vi "labHolo.vi"() -> ()   [LabVIEW 2023] (continued)
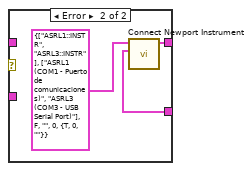
[diagram p2: hidden frame]
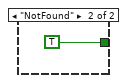
[diagram p4: hidden frame]
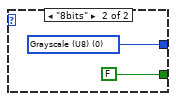
[diagram p5: hidden frame]
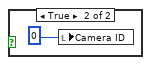
[diagram p6: hidden frame]
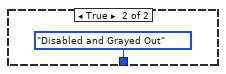
[diagram p7: hidden frame]
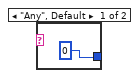
[diagram p13: hidden frame]
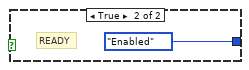
[diagram p14: hidden frame]
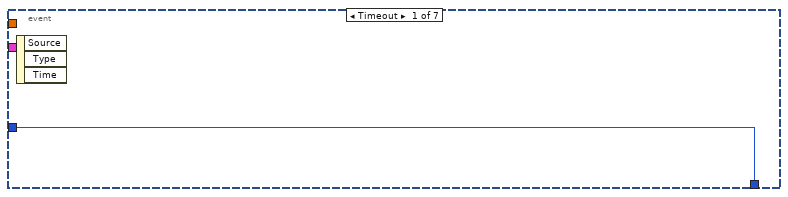
[diagram p15: hidden frame]
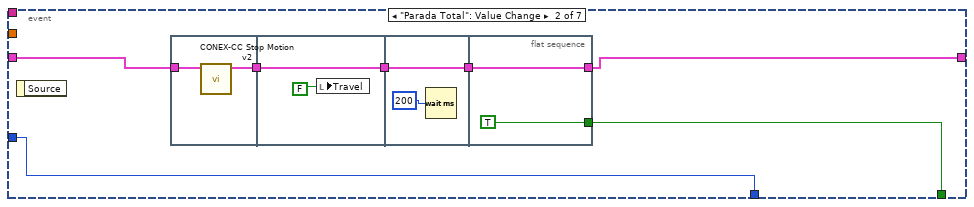
[diagram p16: hidden frame]
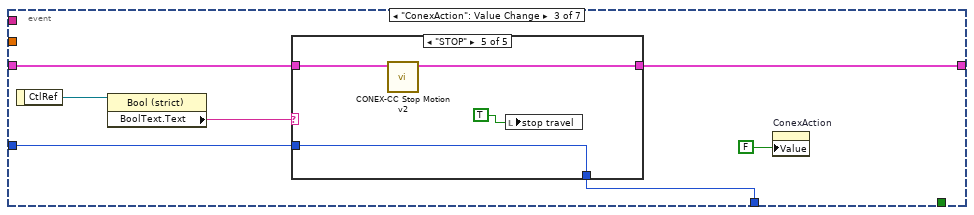
[diagram p17: hidden frame]
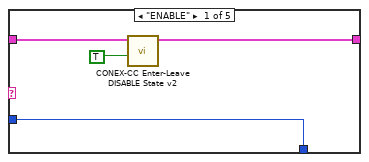
[diagram p18: hidden frame]
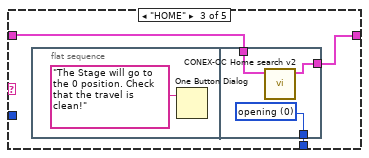
[diagram p20: hidden frame]
            n224 = local write "take reff"(w850) -> ()
            n225 = local write "Mean array"(w851) -> ()
            n226 = local write "Var array"(w851) -> ()
          }
          event "suffix", "Polarizer", "Analyzer", "beam_name", "Save": Value Change {
            n227 = event-data() -> ("CtlRef"=w866:refnum<vi>)  [unwired: 1 in, 5 out]
            n228 = local read "Travel"() -> (w853:bool)
            n229 = property class="Ctl"(reference=w866, error in=w860) -> (reference out=w861:refnum<vi>, error out=w859:errorcluster, "Label.Text"=w865:string)
            n230 = local read "beam_name"() -> (w870:string)
            n231 = local read "paramAux"() -> (w867:string)
            n232 = case shown="True" w853 {
              tunnel: w855 -> [_ w873]
              tunnel: [w871 w872] -> w854
              frame False {
                n233 = local read "suffix"() -> (w871:string)
              }
              frame True {
                n234 = Wait on Notification with Notifier History(0:w873) -> (9:w872:string)  [unwired: 3 in, 3 out]
                n235 = local write "suffix"(w872) -> ()
              }
            }
            n236 = local read "Polarizer"() -> (w869:string)
            n237 = local read "Analyzer"() -> (w868:string)
            n238 = call "getSavePath.vi"("beam_name"=w870, "Polarizer"=w869, "Analyzer"=w868, "prefix"=w867, "suffix"=w854) -> ("appended filename"=w858:string)  [unwired: 10 in]
            n239 = case shown="\"Save\"" w865 {
              tunnel: w858 -> [w874 w891]
              tunnel: w864 -> [_ w893]
              tunnel: w863 -> [_ w892]
              tunnel: [errorcluster {"status"=FALSE, "code"=0, "source"=""} ("error out") w881] -> w862
              tunnel: w861 -> [_ w885]
              tunnel: w859 -> [_ w886]
              tunnel: [w874 w887] -> w856
              tunnel: w853 -> [_ w877]
              frame "Any", Default {
              }
              frame "Save" {
                n240 = property on="Property Node" class="Ctl"(reference=w885, error in=w886, "DisabledEnum"=T11."Disabled and Grayed Out" ("Disabled")) -> (reference out=w884:refnum<vi>, error out=w883:errorcluster)
                n241 = Not(x=w877) -> (.not. x?=w876:bool)
                n242 = local read "Reff ROI"() -> (w889:T8)
                n243 = local read "bit depth"() -> (w888:enum16{"16bits", "14bits", "12bits", "8bits"})
                n244 = property on="CCD Image" class="ImageControl"() -> ("ROI"=w890:T8)  [unwired: 2 in, 2 out]
                n245 = call "saveImage.vi"("UserDialog"=w876, "error in"=w883, "bit depth"=w888, "session in"=w892, "Reff ROI"=w889, "main ROI"=w890, "appended filename"=w891, "Image in"=w893) -> ("error out"=w882:errorcluster, "png filename"=w887:string)  [unwired: 2 out]
                n246 = property on="Property Node" class="Ctl"(reference=w884, error in=w882, "DisabledEnum"=T11."Enabled" ("Disabled"), "Value"=FALSE ("Save")) -> (error out=w881:errorcluster)  [unwired: 1 out]
              }
            }
            n247 = local write "default filename"(w858) -> ()
            n248 = Send Notification(notification=w856, notifier=w857) -> ()  [unwired: 1 in, 2 out]
          }
          event "FPS", "Exposure (ms)", "Gain": Value Change {
            n249 = event-data() -> ("CtlRef"=w902:refnum<vi>, "NewVal"=w905:dbl)  [unwired: 1 in, 4 out]
            n250 = property class="DigNum (strict)"(reference=w902) -> ("Label.Text"=w903:string)  [unwired: 1 in, 2 out]
            n251 = case shown="\"FPS\"" w903 {
              tunnel: w906 -> [w913 w920 w929]
              tunnel: w905 -> [w912 w919 w921]
              tunnel: [w911 w918 w927] -> w904
              tunnel: w895 -> [w908 w917 w922]
              tunnel: [w909 w916 w926] -> w897
              tunnel: [w910 w915 w925] -> w896
              tunnel: w894 -> [w907 w914 w928]
              frame "Exposure (ms)", Default {
                n252 = call "set_exposure.vi"("error in (no error)"=w907, "cam ID"=w908, "exposure"=w912, "Session in"=w913) -> ("error out"=w911:errorcluster, "true FPS"=w909:dbl, "true exposure"=w910:dbl)  [unwired: 3 in, 1 out]
              }
              frame "FPS" {
                n253 = call "set_fps.vi"("error in (no error)"=w914, "cam ID"=w917, "FPS"=w919, "Session in"=w920) -> ("error out"=w918:errorcluster, "true Exposure"=w915:dbl, "true FPS"=w916:dbl)  [unwired: 3 in, 1 out]
              }
              frame "Gain" {
                n254 = local read "gains"() -> (w924:dbl[])
                n255 = call "set_gain.vi"("error in (no error)"=w928, "cam ID"=w922, "Gain"=w921, "Session in"=w929) -> ("error out"=w927:errorcluster, "true Exposure"=w925:dbl, "true FPS"=w926:dbl)  [unwired: 3 in, 1 out]
                n256 = Replace Array Subset(array=w924, new element=w921, index=w922) -> (w923:dbl[])
                n257 = local write "gains"(w923) -> ()
              }
            }
            n258 = local write "Exposure (ms)"(w896) -> ()
            n259 = local write "FPS"(w897) -> ()
            n260 = local read "exposures"() -> (w900:dbl[])
            n261 = local read "FPSs"() -> (w901:dbl[])
            n262 = Replace Array Subset(array=w900, new element=w896, index=w895) -> (w898:dbl[])
            n263 = Replace Array Subset(array=w901, new element=w897, index=w895) -> (w899:dbl[])
            n264 = local write "exposures"(w898) -> ()
            n265 = local write "FPSs"(w899) -> ()
          }
          event "Camera ID": Value Change {
            n266 = event-data() -> ("OldVal"=w931:u16, "NewVal"=w930:u16)  [unwired: 1 in, 4 out]
            n267 = flat-sequence {
              tunnel: w931 -> [w932]
              tunnel: w930 -> [w944]
              frame #0 {
                n268 = local read "Exposure (ms)"() -> (w941:dbl)
                n269 = local read "gains"() -> (w935:dbl[])
                n270 = local read "FPSs"() -> (w936:dbl[])
                n271 = local read "Gain"() -> (w933:dbl)
                n272 = local read "exposures"() -> (w940:dbl[])
                n273 = local read "FPS"() -> (w938:dbl)
                n274 = Replace Array Subset(array=w935, new element=w933, index=w932) -> (w934:dbl[])
                n275 = Replace Array Subset(array=w940, new element=w941, index=w932) -> (w939:dbl[])
                n276 = Replace Array Subset(array=w936, new element=w938, index=w932) -> (w937:dbl[])
                n277 = local write "exposures"(w939) -> ()
                n278 = local write "FPSs"(w937) -> ()
                n279 = local write "gains"(w934) -> ()
              }
              frame #1 {
                n280 = local read "exposures"() -> (w950:dbl[])
                n281 = local read "FPSs"() -> (w949:dbl[])
                n282 = local read "gains"() -> (w943:dbl[])
                n283 = Index Array(array=w949, index=w944) -> (element=w948:dbl)
                n284 = Index Array(array=w950, index=w944) -> (element=w947:dbl)
                n285 = Index Array(array=w943, index=w944) -> (element=w942:dbl)
                n286 = property on="FPS" class="DigNum (strict)"("Val(Sgnl)"=w948) -> (error out=w946:errorcluster)  [unwired: 2 in, 1 out]
                n287 = property on="Exposure (ms)" class="DigNum (strict)"(error in=w946, "Val(Sgnl)"=w947) -> (error out=w945:errorcluster)  [unwired: 1 in, 1 out]
                n288 = property on="Gain" class="DigNum (strict)"(error in=w945, "Val(Sgnl)"=w942) -> ()  [unwired: 1 in, 2 out]
              }
            }
          }
          event "Parada Total": Value Change {
            n289 = event-data() -> ("NewVal"=w951:bool)  [unwired: 1 in, 5 out]
          }
        }
        "py error" <- w804
      }
      n290 = timed-loop {
        timing: w292 -> [_]
        timing-out: [_] -> w291
        shift-right: [w383] -> w290
        shift-left: w289 -> [w389]
        tunnel: w277 -> [w369]
        stop <- w384 stop-if-true
        # "Working loop"
        n291 = node-c288() -> ()  [unwired: 2 out]
        n292 = call "CONEX-CC Get Current Position v2.vi"("Connection Cluster in"=w389) -> ("Current position"=w380:dbl, "Connection Cluster out"=w388:T16)  [unwired: 8 in, 1 out]
        n293 = local read "Travel"() -> (w373:bool)
        n294 = call "CONEX-CC Get Positioner Error And Controller State v2.vi"("Connection Cluster in"=w388) -> ("Controller state"=w386:string, "Positioner error"=w387:string, "Connection Cluster out"=w383:T16)  [unwired: 8 in]
        n295 = Not(x=w373) -> (.not. x?=w374:bool)
        n296 = call "Get Positioner Error And Controller State Descriptions.vi"("Controller state"=w386, "Positioner error"=w387) -> ("Color"=w392:u32, "Action name"=w377:string, "Controller state description"=→"Controller state description":string, "IsReady?"=w372:bool)  [unwired: 2 out]
        "ConexCC ready" <- w372
        n297 = And(x=w374, y=w372) -> (x .and. y?=w375:bool)
        n298 = property on="ConexAction" class="Bool (strict)"("BoolText.Text"=w377) -> ()  [unwired: 2 in, 2 out]
        n299 = property on="Controller state description" class="Str"("Text.FontColor"=w392) -> ()  [unwired: 2 in, 2 out]
        n300 = case shown="False" w375 {
          tunnel: [T11."Disabled and Grayed Out" ("Disabled") T11."Enabled" ("Disabled")] -> w378
          frame False {
            # "MOVING"
          }
          frame True {
            # "READY"
          }
        }
        n301 = String Length(string=w377) -> (length=w391:i32)
        n302 = case shown="\"DISABLE\"" w377 {
          tunnel: [0 2] -> w376
          frame "Any", Default {
          }
          frame "DISABLE" {
          }
        }
        n303 = Greater Than 0?(x=w391) -> (x > 0?=w390:bool)
        n304 = property on="ConexAction" class="Bool (strict)"("DisabledEnum"=w376, "Visible"=w390) -> ()  [unwired: 2 in, 2 out]
        n305 = property on="Go0" class="Bool (strict)"("Disabled"=w378) -> ()  [unwired: 2 in, 2 out]
        n306 = property on="Go1" class="Bool (strict)"("Disabled"=w378) -> ()  [unwired: 2 in, 2 out]
        n307 = property on="Go2" class="Bool (strict)"("Disabled"=w378) -> ()  [unwired: 2 in, 2 out]
        n308 = property on="Units" class="CmbBox"("Disabled"=w378) -> ()  [unwired: 2 in, 2 out]
        n309 = property on="Tare" class="Bool (strict)"("Disabled"=w378) -> ()  [unwired: 2 in, 2 out]
        n310 = property on="Travel" class="Bool (strict)"("Disabled"=w378) -> ()  [unwired: 2 in, 2 out]
        n311 = property on="step forward" class="Bool (strict)"("Disabled"=w378) -> ()  [unwired: 2 in, 2 out]
        n312 = property on="step backward" class="Bool (strict)"("Disabled"=w378) -> ()  [unwired: 2 in, 2 out]
        n313 = property on="SaveTravel" class="Bool (strict)"("Disabled"=w378) -> ()  [unwired: 2 in, 2 out]
        n314 = local read "Units"() -> (w382:string)
        n315 = local read "lambda"() -> (w381:dbl)
        n316 = call "mm2units.vi"("lambda (nm)"=w381, "target units"=w382, "raw position (mm)"=w380) -> ("position in units"=w379:dbl)  [unwired: 8 in]
        n317 = local read "Zero pos."() -> (w385:dbl)
        n318 = local read "Travel"() -> (w371:bool)
        n319 = local write "Raw position"(w379) -> ()
        n320 = Subtract(x=w379, y=w385) -> (x-y=w370:dbl)
        n321 = local write "Relative pos."(w370) -> ()
        n322 = case shown="True" w371 {
          tunnel: w370 -> [_ w395]
          tunnel: w369 -> [_ w394]
          frame False {
          }
          frame True {
            n323 = Send Notification(notification=w395, notifier=w394) -> ()  [unwired: 1 in, 2 out]
          }
        }
        n324 = local read "Parada Total"() -> (w384:bool)
        n325 = node-c288() -> ()  [unwired: 2 out]
      }
      n326 = while {
        tunnel: w295 -> [w523]
        shift-right: [w522] -> _
        shift-left: w294 -> [w521]
        shift-right: [w520] -> _
        shift-left: w296 -> [w524]
        shift-right: [w519] -> _
        shift-left: _ -> [w518]
        shift-right: [w516] -> _
        shift-left: w293 -> [w517]
        stop <- w525 stop-if-true
        # "SLM control"
        # "CGH path"
        # "Theo"
        # "SLM"
        n327 = event shown="[1] \"Radio\", \"Trans\", \"HoloNum\", \"ModType\", \"Semi\", \"Active\", \"paramVal\", \"paramStr\", \"paramAux\", \"Phase\", \"Flip\": Value Change" {
          selector: _ -> [_ _ _ _ _ _ _]
          dyn-events: _ -> [_ _ _ _ _ _ _]
          timeout: _ -> [_ _ _ _ _ _ _]
          tunnel: w517 -> [w526 w540 w608 w661 w717 _ _]
          tunnel: [_ _ _ _ _ _ w793] -> w525
          tunnel: w524 -> [w528 w543 _ _ _ w754 _]
          tunnel: w523 -> [_ _ _ _ _ _ _]
          tunnel: [_ w538 _ _ _ _ _] -> w522
          tunnel: w521 -> [_ w546 _ _ _ _ _]
          tunnel: [w528 w539 _ _ _ w756 _] -> w520
          tunnel: [w527 w541 _ _ _ w755 _] -> w519
          tunnel: w518 -> [w527 w542 _ _ _ w753 _]
          tunnel: [w526 w540 w608 w661 w717 w752 _] -> w516
          event Timeout {
            n328 = event-data() -> ()  [unwired: 1 in, 3 out]
          }
          event "Radio", "Trans", "HoloNum", "ModType", "Semi", "Active", "paramVal", "paramStr", "paramAux", "Phase", "Flip": Value Change {
            # "Display = #item + 1"
            # "Old"
            # "New"
            n329 = event-data() -> ("CtlRef"=w544:refnum<vi>, "OldVal"=w550:variant, "NewVal"=w545:variant)  [unwired: 1 in]
            n330 = case shown="1" w540 {
              tunnel: [w555 w556] -> w552
              frame 0, Default {
                n331 = local read "SLM1 cluster"() -> (w555:T2)
              }
              frame 1 {
                n332 = local read "SLM2 cluster"() -> (w556:T2)
              }
            }
            n333 = property class="Ctl"(reference=w544) -> ("Label.Text"=w551:string)  [unwired: 1 in, 2 out]
            n334 = call "updateHoloBundle.vi"("NewValue"=w545, "input cluster"=w552, "CtlRef"=w544) -> ("output cluster"=w549:T19)  [unwired: 7 in, 1 out]
            n335 = Increment(x=w540) -> (x+1=w548:u16)
            n336 = call "loadShowHolo.vi"("Display"=w548, "error in (no error)"=w546, "prev. path"=w542, "SLM1 cluster"=w549, "Image in"=w543) -> ("error out"=w538:errorcluster, "path exist"=w547:bool, "appended path"=w541:path, "Image out"=w539:T6)  [unwired: 3 in]
            n337 = case shown="\"Radio\"" w551 {
              tunnel: w550 -> [w558 w564 _ w570 _ w581 w587 w593 _ _]
              tunnel: w545 -> [_ _ _ _ w579 _ _ _ w602 w606]
              tunnel: w547 -> [w557 w563 _ w569 _ w580 w586 w592 _ _]
              frame "HoloNum" {
                n338 = case shown="False" w557 {
                  tunnel: w558 -> [w559 _]
                  frame False {
                    n339 = feedback #1() -> (w560:dbl)  [unwired: 1 in]
                    n340 = Variant To Data(type=w560, Variant=w559) -> (data=w562:dbl)  [unwired: 1 in, 1 out]
                    n341 = property on="HoloNum" class="DigNum (strict)"("Value"=w562) -> ("Value"=w561:dbl)  [unwired: 2 in, 2 out]
                    n342 = feedback-in #1(w561) -> ()
                  }
                  frame True {
                  }
                }
              }
              frame "ParamStr" {
                n343 = case shown="False" w563 {
                  tunnel: w564 -> [w565 _]
                  frame False {
                    n344 = feedback #2() -> (w566:string)  [unwired: 1 in]
                    n345 = Variant To Data(type=w566, Variant=w565) -> (data=w568:string)  [unwired: 1 in, 1 out]
                    n346 = property on="paramStr" class="Str"("Value"=w568) -> ("Value"=w567:string)  [unwired: 2 in, 2 out]
                    n347 = feedback-in #2(w567) -> ()
                  }
                  frame True {
                  }
                }
              }
              frame "Any", Default {
              }
              frame "ParamVal" {
                n348 = case shown="False" w569 {
                  tunnel: w570 -> [w571 _]
                  frame False {
                    n349 = feedback #3() -> (w572:i64)  [unwired: 1 in]
                    n350 = Variant To Data(type=w572, Variant=w571) -> (data=w574:i64)  [unwired: 1 in, 1 out]
                    n351 = property on="paramVal" class="DigNum (strict)"("Value"=w574) -> ("Value"=w573:i64)  [unwired: 2 in, 2 out]
                    n352 = feedback-in #3(w573) -> ()
                  }
                  frame True {
                  }
                }
              }
              frame "Active" {
                n353 = Variant To Data(type=0, Variant=w579) -> (data=w575:i32)  [unwired: 1 in, 1 out]
                n354 = Not Equal?(x=u16 0, y=w575) -> (x != y?=w576:bool)
                n355 = property on="Active" class="Ring (strict)"("Blinking"=w576) -> ()  [unwired: 2 in, 2 out]
              }
              frame "ParamAux" {
                n356 = case shown="False" w580 {
                  tunnel: w581 -> [w582 _]
                  frame False {
                    n357 = feedback #4() -> (w583:string)  [unwired: 1 in]
                    n358 = Variant To Data(type=w583, Variant=w582) -> (data=w585:string)  [unwired: 1 in, 1 out]
                    n359 = property on="paramAux" class="Str"("Value"=w585) -> ("Value"=w584:string)  [unwired: 2 in, 2 out]
                    n360 = feedback-in #4(w584) -> ()
                  }
                  frame True {
                  }
                }
              }
              frame "ModType" {
                n361 = case shown="False" w586 {
                  tunnel: w587 -> [w589 _]
                  frame False {
                    n362 = feedback #5() -> (w591:string)  [unwired: 1 in]
                    n363 = Variant To Data(type=w591, Variant=w589) -> (data=w588:string)  [unwired: 1 in, 1 out]
                    n364 = property on="ModType" class="CmbBox"("Value"=w588) -> ("Value"=w590:string)  [unwired: 2 in, 2 out]
                    n365 = feedback-in #5(w590) -> ()
                  }
                  frame True {
                  }
                }
              }
              frame "Radio" {
                n366 = case shown="False" w592 {
                  tunnel: w593 -> [w596 _]
                  frame False {
                    n367 = Variant To Data(type=0, Variant=w596) -> (data=w594:i32)  [unwired: 1 in, 1 out]
                    n368 = local write "Radio"(w594) -> ()
                  }
                  frame True {
                  }
                }
              }
              frame "Trans" {
                n369 = Variant To Data(type=0.0, Variant=w602) -> (data=w600:dbl)  [unwired: 1 in, 1 out]
                n370 = call "transAndPhaseManager.vi"("Trans in"=w600) -> ("Trans %"=w599:dbl, "Intensity"=w598:dbl, "T gl"=w597:dbl)  [unwired: 10 in, 2 out]
                n371 = local write "T%"(w599) -> ()
                n372 = local write "Int"(w598) -> ()
                n373 = local write "Tgl"(w597) -> ()
              }
              frame "Phase" {
                n374 = Variant To Data(type=0.0, Variant=w606) -> (data=w603:dbl)  [unwired: 1 in, 1 out]
                n375 = call "transAndPhaseManager.vi"("Phase in"=w603) -> ("Phase Deg"=w605:dbl, "Phase Rad"=w604:dbl)  [unwired: 10 in, 3 out]
                n376 = local write "PhDeg"(w605) -> ()
                n377 = local write "PhRad"(w604) -> ()
              }
            }
            n378 = case shown="1" w540 {
              tunnel: w549 -> [w553 w554]
              frame 0, Default {
                n379 = local write "SLM1 cluster"(w553) -> ()
              }
              frame 1 {
                n380 = local write "SLM2 cluster"(w554) -> ()
              }
            }
            n381 = local read "Radio"() -> (w530:T7)
            n382 = local read "Active"() -> (w537:u16)
            n383 = call "enableDisableSLMbuttons.vi"("Active"=w537, "Radio"=w530) -> ("Semi"=w532:T11, "ModType"=w533:T11, "Phase"=w534:T11, "Trans"=w535:T11, "HoloCode"=w531:T11, "PrefabrHolo"=w536:T11, "just ON/OFF"=w529:T11)  [unwired: 3 in]
            n384 = property on="Flip" class="CmbBox"("DisabledEnum"=w529) -> ()  [unwired: 2 in, 2 out]
            n385 = property on="Radio" class="RadioBtnsControl (strict)"("DisabledEnum"=w529) -> ()  [unwired: 2 in, 2 out]
            n386 = property on="HoloNum" class="DigNum (strict)"("DisabledEnum"=w536) -> ()  [unwired: 2 in, 2 out]
            n387 = property on="paramAux" class="Str"("DisabledEnum"=w536) -> ()  [unwired: 2 in, 2 out]
            n388 = property on="Xoffset" class="DigNum (strict)"("DisabledEnum"=w529) -> ()  [unwired: 2 in, 2 out]
            n389 = property on="Sync SLMs" class="Bool"("DisabledEnum"=w529) -> ()  [unwired: 2 in, 2 out]
            n390 = property on="ModType" class="CmbBox"("DisabledEnum"=w533) -> ()  [unwired: 2 in, 2 out]
            n391 = property on="Trans" class="Slide (strict)"("DisabledEnum"=w535) -> ()  [unwired: 2 in, 2 out]
            n392 = property on="setXi" class="Bool (strict)"("DisabledEnum"=w529) -> ()  [unwired: 2 in, 2 out]
            n393 = property on="paramStr" class="Str"("DisabledEnum"=w536) -> ()  [unwired: 2 in, 2 out]
            n394 = property on="paramVal" class="DigNum (strict)"("DisabledEnum"=w536) -> ()  [unwired: 2 in, 2 out]
            n395 = property on="Yoffset" class="DigNum (strict)"("DisabledEnum"=w529) -> ()  [unwired: 2 in, 2 out]
            n396 = property on="XYswap" class="Ring (strict)"("DisabledEnum"=w529) -> ()  [unwired: 2 in, 2 out]
            n397 = property on="Phase" class="Slide (strict)"("DisabledEnum"=w534) -> ()  [unwired: 2 in, 2 out]
            n398 = property on="T%" class="DigNum (strict)"("DisabledEnum"=w535) -> ()  [unwired: 2 in, 2 out]
            n399 = property on="setXf" class="Bool (strict)"("DisabledEnum"=w529) -> ()  [unwired: 2 in, 2 out]
            n400 = property on="Xgros" class="Slide (strict)"("DisabledEnum"=w529) -> ()  [unwired: 2 in, 2 out]
            n401 = property on="Semi" class="Bool (strict)"("DisabledEnum"=w532) -> ()  [unwired: 2 in, 2 out]
            n402 = property on="Xreverse" class="Ring (strict)"("DisabledEnum"=w529) -> ()  [unwired: 2 in, 2 out]
            n403 = property on="PhDeg" class="DigNum (strict)"("DisabledEnum"=w534) -> ()  [unwired: 2 in, 2 out]
            n404 = property on="setYi" class="Bool (strict)"("DisabledEnum"=w529) -> ()  [unwired: 2 in, 2 out]
            n405 = property on="Tgl" class="DigNum (strict)"("DisabledEnum"=w535) -> ()  [unwired: 2 in, 2 out]
            n406 = property on="Ygros" class="Slide (strict)"("DisabledEnum"=w529) -> ()  [unwired: 2 in, 2 out]
            n407 = property on="Yreverse" class="Ring (strict)"("DisabledEnum"=w529) -> ()  [unwired: 2 in, 2 out]
            n408 = property on="setYf" class="Bool (strict)"("DisabledEnum"=w529) -> ()  [unwired: 2 in, 2 out]
            n409 = property on="PhRad" class="DigNum (strict)"("DisabledEnum"=w534) -> ()  [unwired: 2 in, 2 out]
            n410 = property on="Int" class="DigNum (strict)"("DisabledEnum"=w535) -> ()  [unwired: 2 in, 2 out]
            n411 = property on="Xfine" class="Slide (strict)"("DisabledEnum"=w529) -> ()  [unwired: 2 in, 2 out]
            n412 = property on="help code" class="Bool"("DisabledEnum"=w531) -> ()  [unwired: 2 in, 2 out]
            n413 = property on="HoloCode" class="Str"("DisabledEnum"=w531) -> ()  [unwired: 2 in, 2 out]
            n414 = property on="doCenter" class="Bool (strict)"("DisabledEnum"=w529) -> ()  [unwired: 2 in, 2 out]
            n415 = property on="Yfine" class="Slide (strict)"("DisabledEnum"=w529) -> ()  [unwired: 2 in, 2 out]
          }
          event "Xoffset", "Yoffset", "Xgros", "Ygros", "Xfine", "Yfine", "doCenter": Value Change {
            n416 = event-data() -> ("CtlRef"=w611:refnum<vi>, "NewVal"=w610:variant)  [unwired: 1 in, 4 out]
            n417 = local write "doCenter"(FALSE ("doCenter")) -> ()
            n418 = case shown="1" w608 {
              tunnel: [w620 w621] -> w612
              frame 0, Default {
                n419 = local read "1_posCluster"() -> (w620:T4)
              }
              frame 1 {
                n420 = local read "2_posCluster"() -> (w621:T4)
              }
            }
            n421 = property class="Ctl"(reference=w611) -> ("Label.Text"=w616:string)  [unwired: 1 in, 2 out]
            n422 = case shown="\"doCenter\"" w616 {
              tunnel: w612 -> [w626 w631 w636 w641 w646 w651 w655 w660]
              tunnel: w610 -> [w625 w630 w635 w640 w645 w650 _ _]
              tunnel: [w622 w627 w632 w637 w642 w647 w654 w660] -> w617
              frame "Xoffset" {
                n423 = Variant To Data(type=0.0, Variant=w625) -> (data=w624:dbl)  [unwired: 1 in, 1 out]
                n424 = Bundle By Name(cluster=w626, "1_Xoffset"=w624) -> (w622:T4)
              }
              frame "Yoffset" {
                n425 = Variant To Data(type=0.0, Variant=w630) -> (data=w628:dbl)  [unwired: 1 in, 1 out]
                n426 = Bundle By Name(cluster=w631, "1_Yoffset"=w628) -> (w627:T4)
              }
              frame "Xgros" {
                n427 = Variant To Data(type=0.0, Variant=w635) -> (data=w633:dbl)  [unwired: 1 in, 1 out]
                n428 = Bundle By Name(cluster=w636, "1_Xgros"=w633) -> (w632:T4)
              }
              frame "Ygros" {
                n429 = Variant To Data(type=0.0, Variant=w640) -> (data=w638:dbl)  [unwired: 1 in, 1 out]
                n430 = Bundle By Name(cluster=w641, "1_Ygros"=w638) -> (w637:T4)
              }
              frame "Xfine" {
                n431 = Variant To Data(type=0.0, Variant=w645) -> (data=w643:dbl)  [unwired: 1 in, 1 out]
                n432 = Bundle By Name(cluster=w646, "1_Xfine"=w643) -> (w642:T4)
              }
              frame "Yfine" {
                n433 = Variant To Data(type=0.0, Variant=w650) -> (data=w648:dbl)  [unwired: 1 in, 1 out]
                n434 = Bundle By Name(cluster=w651, "1_Yfine"=w648) -> (w647:T4)
              }
              frame "doCenter" {
                n435 = local read "Xcenter"() -> (w659:dbl)
                n436 = local read "Ycenter"() -> (w657:dbl)
                n437 = local read "Xpos"() -> (w658:i32)
                n438 = local read "Ypos"() -> (w656:i32)
                n439 = call "centerHolo.vi"("posCluster"=w655, "Ypos"=w656, "Ycenter"=w657, "Xpos"=w658, "Xcenter"=w659) -> ("new Y gros"=w652:dbl, "new X gros"=w653:dbl)  [unwired: 4 in]
                n440 = Bundle By Name(cluster=w655, "1_Xgros"=w653, "1_Ygros"=w652) -> (w654:T4)
                n441 = local write "Xgros"(w653) -> ()
                n442 = local write "Ygros"(w652) -> ()
              }
              frame "Any", Default {
              }
            }
            n443 = case shown="1" w608 {
              tunnel: w617 -> [w618 w619]
              frame 0, Default {
                n444 = local write "1_posCluster"(w618) -> ()
              }
              frame 1 {
                n445 = local write "2_posCluster"(w619) -> ()
              }
            }
            n446 = Increment(x=w608) -> (x+1=w615:u16)
            n447 = call "positionManager.vi"("Display"=w615, "Cluster"=w617) -> ("Y position out"=w614:i32, "X position out"=w613:i32)  [unwired: 5 in, 1 out]
            n448 = local write "Xpos"(w613) -> ()
            n449 = local write "Ypos"(w614) -> ()
          }
          event "Xreverse", "Yreverse", "XYswap": Value Change {
            n450 = event-data() -> ("CtlRef"=w662:refnum<vi>, "NewVal"=w663:u16)  [unwired: 1 in, 4 out]
            n451 = case shown="1" w661 {
              tunnel: [w674 w676] -> w665
              tunnel: [w673 w675] -> w667
              frame 0, Default {
                n452 = local read "1_posCluster"() -> (w674:T4)
                n453 = local read "1_mainPos"() -> (w673:T3)
              }
              frame 1 {
                n454 = local read "2_posCluster"() -> (w676:T4)
                n455 = local read "2_mainPos"() -> (w675:T3)
              }
            }
            n456 = property class="Ring (strict)"(reference=w662) -> ("Label.Text"=w664:string)  [unwired: 1 in, 2 out]
            n457 = case shown="\"XYswap\"" w664 {
              tunnel: [w694 w696 w706 w709] -> w666
              tunnel: w665 -> [w693 w696 w705 w710]
              tunnel: w663 -> [w687 _ w698 w708]
              tunnel: w667 -> [w681 w695 w697 w707]
              tunnel: [w680 w695 w697 w707] -> w668
              frame "XYswap" {
                n458 = Unbundle By Name(w693) -> ("1_Xoffset"=w690:dbl, "1_Yoffset"=w692:dbl, "1_Xgros"=w689:dbl, "1_Ygros"=w691:dbl, "1_Xfine"=w688:dbl, "1_Yfine"=w679:dbl)
                n459 = Unbundle By Name(w681) -> ("1_Xcenter"=w678:dbl, "1_Ycenter"=w677:dbl)
                n460 = local write "Xcenter"(w677) -> ()
                n461 = local write "Ycenter"(w678) -> ()
                n462 = property on="Xoffset" class="DigNum (strict)"("Val(Sgnl)"=w692) -> (error out=w686:errorcluster)  [unwired: 2 in, 1 out]
                n463 = Bundle By Name(cluster=w693, "1_XYswap"=w687, "1_Xoffset"=w692, "1_Yoffset"=w690, "1_Xgros"=w691, "1_Ygros"=w689, "1_Xfine"=w679, "1_Yfine"=w688) -> (w694:T4)
                n464 = Bundle By Name(cluster=w681, "1_Ycenter"=w678, "1_Xcenter"=w677) -> (w680:T3)
                n465 = property on="Yoffset" class="DigNum (strict)"(error in=w686, "Val(Sgnl)"=w690) -> (error out=w683:errorcluster)  [unwired: 1 in, 1 out]
                n466 = property on="Xgros" class="Slide (strict)"(error in=w683, "Val(Sgnl)"=w691) -> (error out=w685:errorcluster)  [unwired: 1 in, 1 out]
                n467 = property on="Ygros" class="Slide (strict)"(error in=w685, "Val(Sgnl)"=w689) -> (error out=w682:errorcluster)  [unwired: 1 in, 1 out]
                n468 = property on="Xfine" class="Slide (strict)"(error in=w682, "Val(Sgnl)"=w679) -> (error out=w684:errorcluster)  [unwired: 1 in, 1 out]
                n469 = property on="Yfine" class="Slide (strict)"(error in=w684, "Val(Sgnl)"=w688) -> ()  [unwired: 1 in, 2 out]
              }
              frame "Any", Default {
              }
              frame "Xreverse" {
                w702 = -1
                n470 = Unbundle By Name(w705) -> ("1_Xgros"=w703:dbl, "1_Xfine"=w704:dbl)
                n471 = Multiply(x=w702, y=w703) -> (x*y=w701:dbl)
                n472 = Multiply(x=w704, y=w702) -> (x*y=w699:dbl)
                n473 = property on="Xgros" class="Slide (strict)"("Val(Sgnl)"=w701) -> (error out=w700:errorcluster)  [unwired: 2 in, 1 out]
                n474 = Bundle By Name(cluster=w705, "1_Xgros"=w701, "1_Xfine"=w699, "1_Xreverse"=w698) -> (w706:T4)
                n475 = property on="Xfine" class="Slide (strict)"(error in=w700, "Val(Sgnl)"=w699) -> ()  [unwired: 1 in, 2 out]
              }
              frame "Yreverse" {
                w714 = -1
                n476 = Unbundle By Name(w710) -> ("1_Ygros"=w715:dbl, "1_Yfine"=w716:dbl)
                n477 = Multiply(x=w714, y=w715) -> (x*y=w713:dbl)
                n478 = Multiply(x=w716, y=w714) -> (x*y=w711:dbl)
                n479 = property on="Ygros" class="Slide (strict)"("Val(Sgnl)"=w713) -> (error out=w712:errorcluster)  [unwired: 2 in, 1 out]
                n480 = Bundle By Name(cluster=w710, "1_Ygros"=w713, "1_Yfine"=w711, "1_Yreverse"=w708) -> (w709:T4)
                n481 = property on="Yfine" class="Slide (strict)"(error in=w712, "Val(Sgnl)"=w711) -> ()  [unwired: 1 in, 2 out]
              }
            }
            n482 = case shown="0, Default" w661 {
              tunnel: w666 -> [w670 w672]
              tunnel: w668 -> [w669 w671]
              frame 0, Default {
                n483 = local write "1_posCluster"(w670) -> ()
                n484 = local write "1_mainPos"(w669) -> ()
              }
              frame 1 {
                n485 = local write "2_posCluster"(w672) -> ()
                n486 = local write "2_mainPos"(w671) -> ()
              }
            }
          }
          event "setXi", "setXf", "setYi", "setYf": Value Change {
            w719 = FALSE ("setYf")
            n487 = event-data() -> ("CtlRef"=w718:refnum<vi>)  [unwired: 1 in, 5 out]
            n488 = case shown="0, Default" w717 {
              tunnel: [w735 w736] -> w721
              frame 0, Default {
                n489 = local read "1_mainPos"() -> (w735:T3)
              }
              frame 1 {
                n490 = local read "2_mainPos"() -> (w736:T3)
              }
            }
            n491 = property class="Bool (strict)"(reference=w718) -> ("Label.Text"=w720:string)  [unwired: 1 in, 2 out]
            n492 = local read "Ypos"() -> (w723:i32)
            n493 = local read "Xpos"() -> (w722:i32)
            n494 = case shown="\"setYf\"" w720 {
              tunnel: w721 -> [w739 w742 w744 w747 w750]
              tunnel: [w739 w741 w743 w746 w749] -> w724
              tunnel: w722 -> [_ w740 w745 _ _]
              tunnel: w723 -> [_ _ _ w748 w751]
              frame "Any", Default {
              }
              frame "setXi" {
                n495 = Bundle By Name(cluster=w742, "1_Xi"=w740) -> (w741:T3)
              }
              frame "setXf" {
                n496 = Bundle By Name(cluster=w744, "1_Xf"=w745) -> (w743:T3)
              }
              frame "setYi" {
                n497 = Bundle By Name(cluster=w747, "1_Yi"=w748) -> (w746:T3)
              }
              frame "setYf" {
                n498 = Bundle By Name(cluster=w750, "1_Yf"=w751) -> (w749:T3)
              }
            }
            n499 = Unbundle By Name(w724) -> ("1_Xi"=w726:dbl, "1_Xf"=w727:dbl, "1_Yi"=w728:dbl, "1_Yf"=w729:dbl)
            n500 = local write "setYf"(w719) -> ()
            n501 = local write "setYi"(w719) -> ()
            n502 = local write "setXf"(w719) -> ()
            n503 = local write "setXi"(w719) -> ()
            n504 = call "pos2centerRadi.vi"("pos fin"=w727, "pos init"=w726) -> ("semi diff (r)"=w733:dbl, "semi sum (C)"=w734:dbl)  [unwired: 8 in]
            n505 = call "pos2centerRadi.vi"("pos fin"=w729, "pos init"=w728) -> ("semi diff (r)"=w731:dbl, "semi sum (C)"=w732:dbl)  [unwired: 8 in]
            n506 = Divide(x=w733, y=w731) -> (x/y=w730:dbl)
            n507 = Bundle By Name(cluster=w724, "1_Xcenter"=w734, "1_Diam. X"=w733, "1_Ycenter"=w732, "1_Diam. Y"=w731, "1_Form fa."=w730) -> (w725:T3)
            n508 = local write "Form fa."(w730) -> ()
            n509 = local write "Diam. Y"(w731) -> ()
            n510 = local write "Ycenter"(w732) -> ()
            n511 = local write "Diam. X"(w733) -> ()
            n512 = local write "Xcenter"(w734) -> ()
            n513 = case shown="0, Default" w717 {
              tunnel: w725 -> [w737 w738]
              frame 0, Default {
                n514 = local write "1_mainPos"(w737) -> ()
              }
              frame 1 {
                n515 = local write "2_mainPos"(w738) -> ()
              }
            }
          }
          event "SLM_number": Value Change {
            n516 = event-data() -> ("NewVal"=w752:u16)  [unwired: 1 in]
            n517 = case shown="1" w752 {
              tunnel: [w789 w792] -> w784
              tunnel: [w788 w791] -> w768
              tunnel: [w787 w790] -> w778
              frame 0, Default {
                n518 = local read "1_posCluster"() -> (w788:T4)
                n519 = local read "SLM1 cluster"() -> (w789:T2)
                n520 = local read "1_mainPos"() -> (w787:T3)
              }
              frame 1 {
                n521 = local read "SLM2 cluster"() -> (w792:T2)
                n522 = local read "2_posCluster"() -> (w791:T4)
                n523 = local read "2_mainPos"() -> (w790:T3)
              }
            }
            n524 = Unbundle By Name(w784) -> ("1_Radio"=w757:T7, "1_Trans"=w758:dbl, "1_Phase"=w759:dbl, "1_HoloCode"=w760:string, "1_Semi"=w761:bool, "1_Active"=w786:u16, "1_ModType"=w762:string, "1_Flip"=w763:string, "1_HoloNum"=w764:dbl, "1_paramStr"=w765:string, "1_paramVal"=w766:i64, "1_paramAux"=w767:string)
            n525 = Unbundle By Name(w778) -> ("1_Xcenter"=w779:dbl, "1_Ycenter"=w780:dbl, "1_Diam. X"=w781:dbl, "1_Diam. Y"=w782:dbl, "1_Form fa."=w783:dbl)
            n526 = Unbundle By Name(w768) -> ("1_Xoffset"=w769:dbl, "1_Yoffset"=w770:dbl, "1_Xgros"=w771:dbl, "1_Ygros"=w772:dbl, "1_Xfine"=w773:dbl, "1_Yfine"=w774:dbl, "1_Xreverse"=w775:u16, "1_Yreverse"=w776:u16, "1_XYswap"=w777:u16)
            n527 = local write "Radio"(w757) -> ()
            n528 = local write "Trans"(w758) -> ()
            n529 = local write "Phase"(w759) -> ()
            n530 = local write "HoloCode"(w760) -> ()
            n531 = local write "Semi"(w761) -> ()
            n532 = local write "Active"(w786) -> ()
            n533 = local write "ModType"(w762) -> ()
            n534 = local write "Flip"(w763) -> ()
            n535 = local write "HoloNum"(w764) -> ()
            n536 = local write "paramStr"(w765) -> ()
            n537 = local write "paramVal"(w766) -> ()
            n538 = local write "paramAux"(w767) -> ()
            n539 = local write "Xreverse"(w775) -> ()
            n540 = local write "Yreverse"(w776) -> ()
            n541 = local write "XYswap"(w777) -> ()
            n542 = local write "Xcenter"(w779) -> ()
            n543 = local write "Ycenter"(w780) -> ()
            n544 = local write "Diam. X"(w781) -> ()
            n545 = local write "Diam. Y"(w782) -> ()
            n546 = local write "Form fa."(w783) -> ()
            n547 = local write "Xoffset"(w769) -> ()
            n548 = local write "Ygros"(w772) -> ()
            n549 = local write "Xfine"(w773) -> ()
            n550 = local write "Yoffset"(w770) -> ()
            n551 = local write "Xgros"(w771) -> ()
            n552 = local write "Yfine"(w774) -> ()
            n553 = Increment(x=w752) -> (x+1=w785:u16)
            n554 = call "holoPathEditor.vi"("Display"=w785, "prev. Path"=w753, "input cluster"=w784) -> ("appended path"=w755:path)  [unwired: 5 in, 3 out]
            n555 = call "IMAQ ReadFile"("File Path"=w755, "Image"=w754) -> ("Image Out"=w756:T6)  [unwired: 5 in, 4 out]
            n556 = property on="Active" class="Ring (strict)"("Val(Sgnl)"=w786) -> ()  [unwired: 2 in, 2 out]
          }
          event "Parada Total": Value Change {
            n557 = event-data() -> ("NewVal"=w793:bool)  [unwired: 1 in, 5 out]
          }
        }
        n558 = local write "CGH path"(w519) -> ()
        n559 = local write "CGH"(w520) -> ()
        n560 = local write "SLM"(w520) -> ()
        "error get holo" <- w521
      }
      n561 = node-c288(w291) -> ()  [unwired: 1 out]
    }
    frame #3 {
      w956 = FALSE ("Visible")
      n562 = Unbundle By Name(w958) -> ("VISA resource name"=w960:refnum<visa-resource-name>, "error"=w959:errorcluster)
      n563 = Release Notifier(notifier=w954) -> ()  [unwired: 2 in, 3 out]
      n564 = Release Notifier(notifier=w952) -> ()  [unwired: 2 in, 3 out]
      n565 = Release Notifier(notifier=w953) -> (error out=→"error out  (Notifier)":errorcluster)  [unwired: 2 in, 2 out]
      n566 = Release Notifier(notifier=w955) -> ()  [unwired: 2 in, 3 out]
      n567 = property on="Parada Total" class="Bool (strict)"("Value"=FALSE ("Parada Total")) -> ()  [unwired: 2 in, 2 out]
      n568 = call "IMAQ WindClose"("Close All Windows (False)"=TRUE) -> ()  [unwired: 5 in, 1 out]
      n569 = property on="stop travel" class="Bool (strict)"("Visible"=w956, "Value"=w956) -> ()  [unwired: 2 in, 2 out]
      n570 = call <vilib>:"Simple Error Handler.vi"("error in (no error)"=w959) -> ()  [unwired: 1 in, 8 out]
      n571 = call "_Close Communications.vi"("Instrument Channel"=w960) -> ()  [unwired: 14 in, 1 out]
    }
  }
